vi "MPS_Mag_Core.vi"(0 "EmptyBoreBaseline_Mag_BMon":dbl[](array[numeric])=array[420000 elements], 5 "EmptyBoreBaseline_Mag":dbl[](array[numeric])=array[420000 elements]) -> (1 "Samples Per Acquisition":dbl=21000.0, 3 "Drive IMon":waveform(dbl), 4 "Susceptibility Curves":cluster{"Y":dbl[], "Y":dbl[]}[](graph), 6 "Rx Smooth":dbl[](graph), 10 "BMon_Smooth":dbl[](graph), 12 "Bias Current":waveform(dbl)(graph)={"t0"=timestamp(3727906504.0247726 s since 1904-01-01), "dt"=9.9999999999997e-07, "Y"=array[420000 elements], "attributes"=variant("NI_ChannelName"=variant(string "H1/ai5"), "NI_UnitDescription"=variant(string "Volts"))}, 13 "Rx_Raw":waveform(dbl), 14 "RxBaselineSub":waveform(dbl)(graph), 15 "Bias Smooth":dbl[](graph))   [LabVIEW 2021]
uses:
  <vilib>/Analysis/baseanly.llb/Mean (DBL).vi
  <extravilib>/ChannelInstances/Tag-dbl/Write With Abort.vi
  MPS_global_variables.vi
  <extravilib>/ChannelInstances/Tag-dbl/Instantiate.vi
  <extravilib>/ChannelInstances/Tag-dbl/Endpoint.vi
  <extravilib>/ChannelInstances/Tag-dbl.lvlib
  <vilib>/Analysis/NI_AALBase.lvlib
panel:
  out "Bias Current Amps":waveform(dbl)(graph)={"t0"=timestamp(3727906504.0247726 s since 1904-01-01), "dt"=9.9999999999997e-07, "Y"=array[420000 elements], "attributes"=variant("NI_ChannelName"=variant(string "H1/ai5"), "NI_UnitDescription"=variant(string "Volts"))}
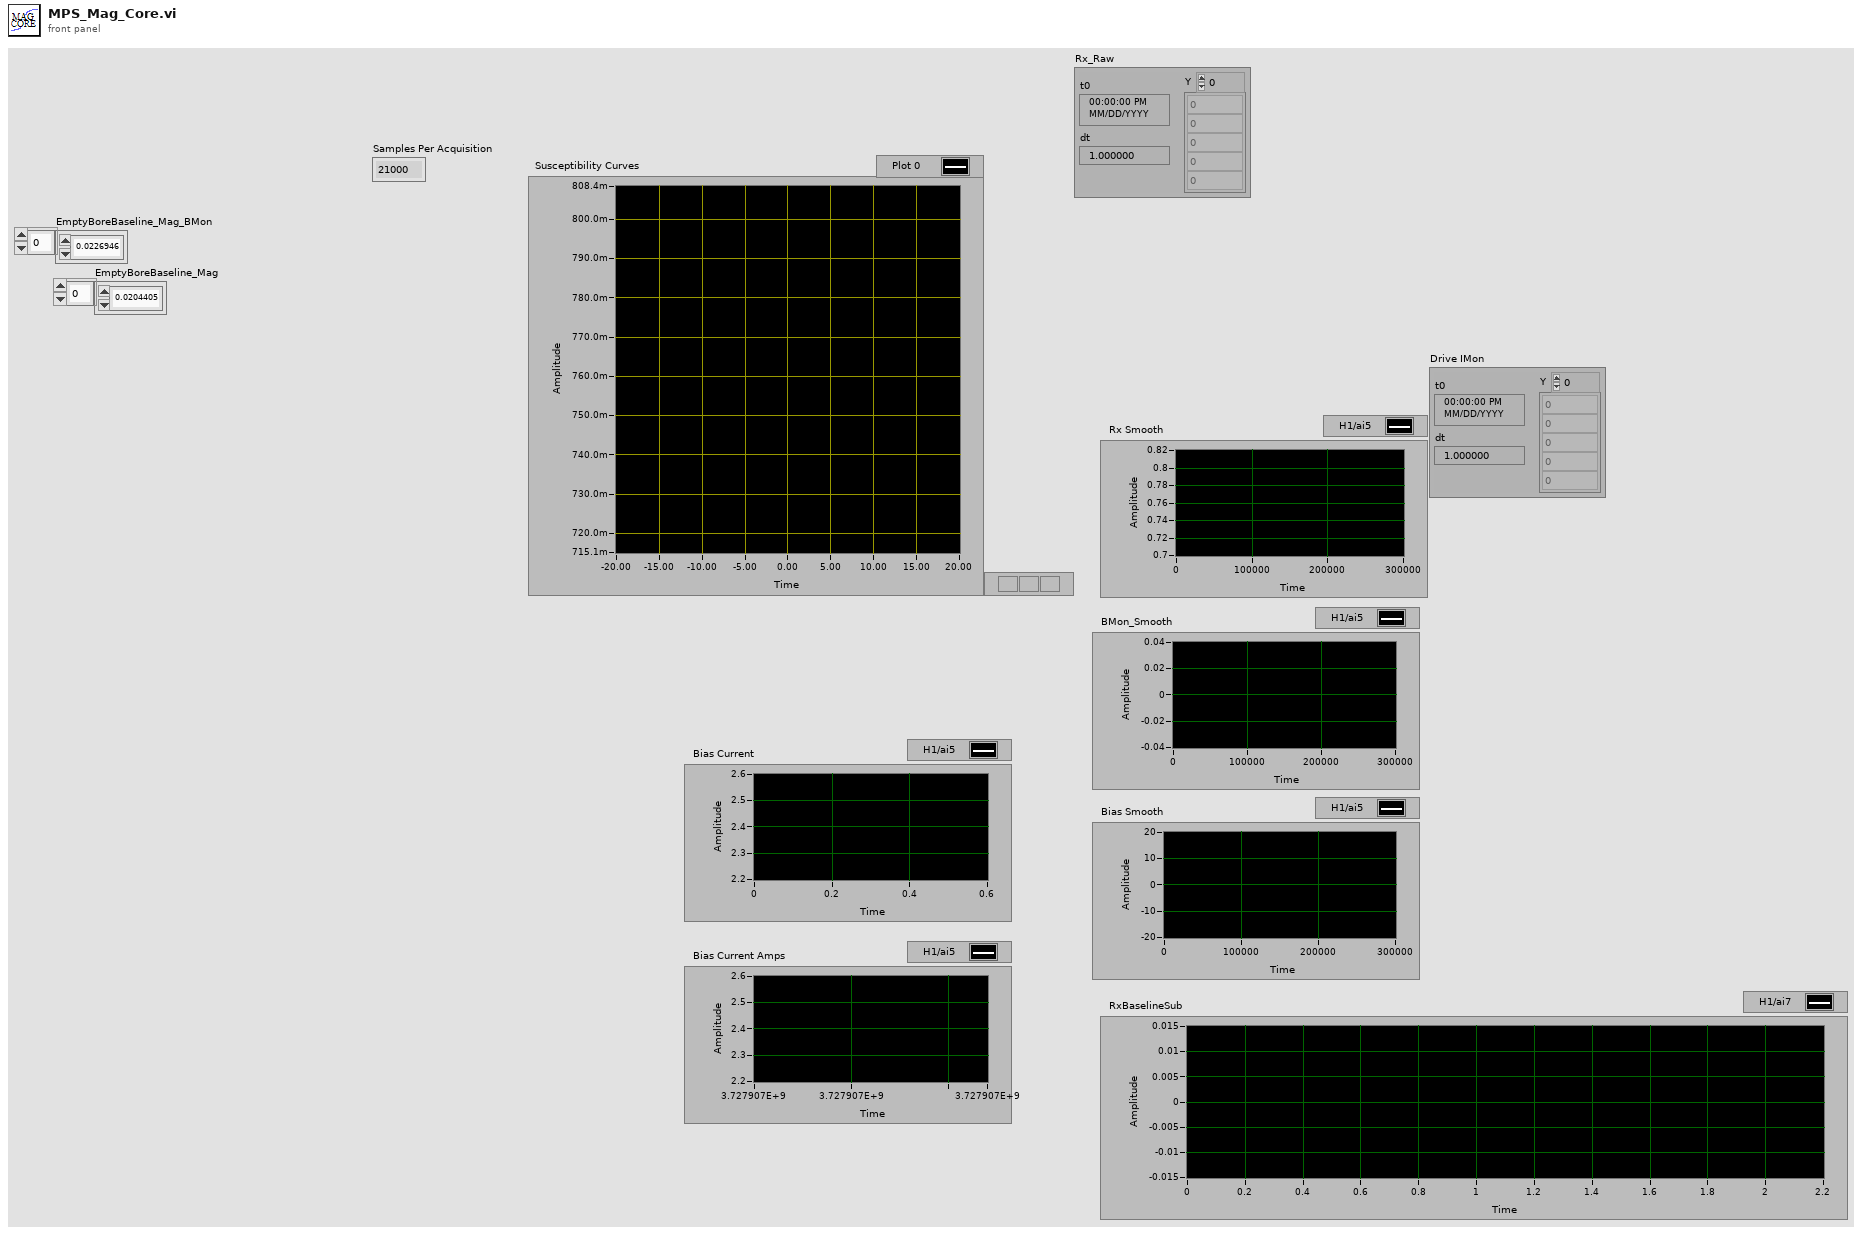
[diagram p1: front panel]
types:
  T1 = typedef "Tag-dbl.lvlib/))Channel.ctl" = refnum<queue>
  T2 = cluster{"sample rate":dbl, "Tx freq":dbl, "Tx amp":dbl, "Tx cycles\nSpectroscopy":dbl, "Bias amp":dbl, "Bias freq":dbl, "Receive range":dbl, "Bias Periods\nMagnetometry":dbl, "Tx Freq Division Factor":dbl, "Drive Periods per Bias":dbl, "TX harmonics":dbl[]}
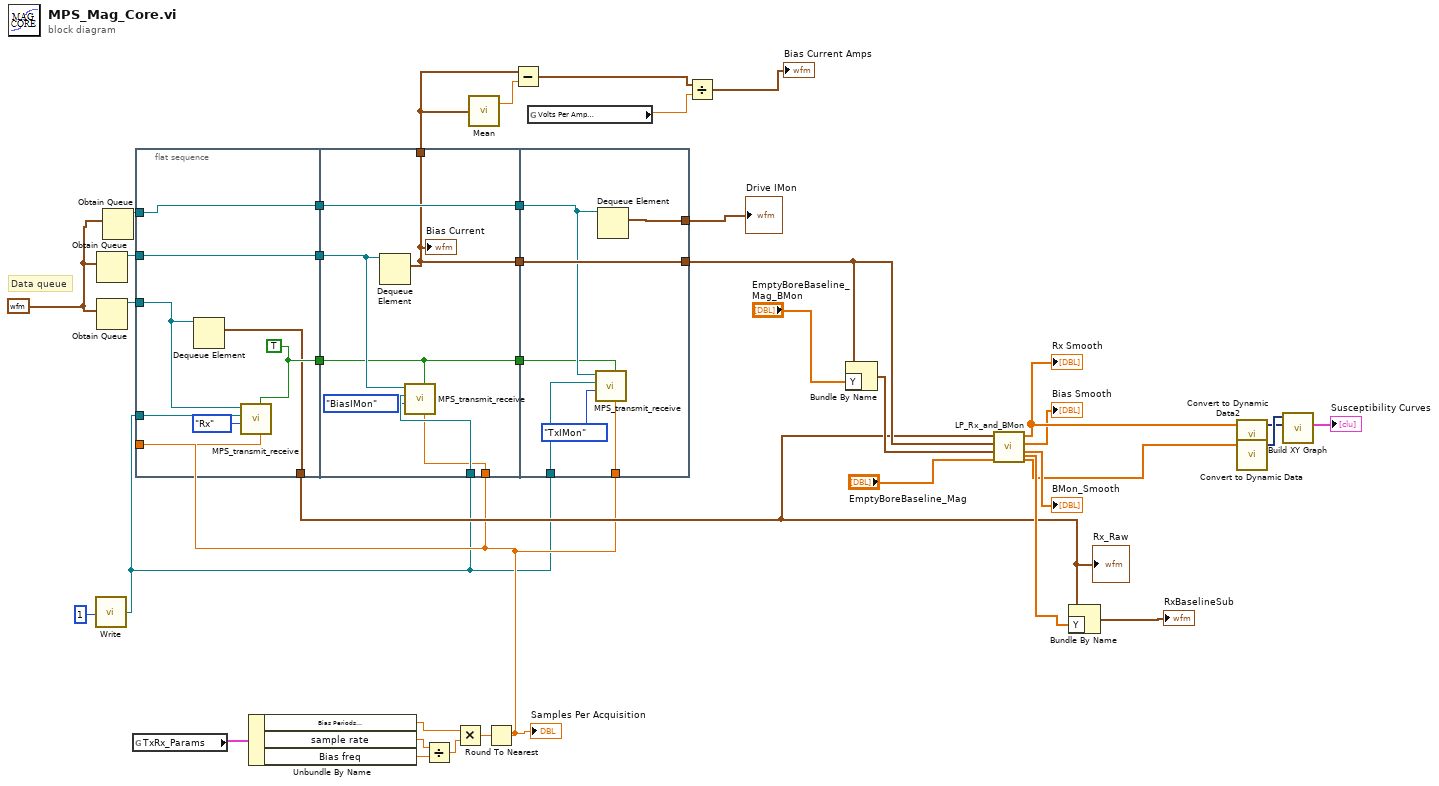
[diagram p0: block diagram]
diagram:
  w14 = waveform(dbl) {"t0"=timestamp(0 s since 1904-01-01), "dt"=1.0, "Y"=[]} ("Waveform")
  # "Data queue"
  n1 = call <extravilib>:"Write.vi"("element"=1 ("number of readouts")) -> ("channel"=w8:T1)  [unwired: 1 out]
  n2 = Obtain Queue(element data type=w14) -> (queue out=w35:refnum<queue>)  [unwired: 4 in, 2 out]
  n3 = Obtain Queue(element data type=w14) -> (queue out=w36:refnum<queue>)  [unwired: 4 in, 2 out]
  n4 = Obtain Queue(element data type=w14) -> (queue out=w11:refnum<queue>)  [unwired: 4 in, 2 out]
  n5 = global read "MPS_global_variables.vi" "TxRx_Params"() -> (w29:T2)
  n6 = flat-sequence {
    tunnel: w36 -> [w46]
    tunnel: [w45] -> w39
    tunnel: w8 -> [w47]
    tunnel: w35 -> [w45]
    tunnel: [w42] -> w16
    tunnel: w9 -> [w44]
    tunnel: [w43] -> w38
    tunnel: [w41] -> w12
    tunnel: w11 -> [w41]
    tunnel: w39 -> [w54]
    tunnel: w8 -> [w53]
    tunnel: w9 -> [w52]
    tunnel: w38 -> [w49]
    tunnel: [w48] -> w15
    tunnel: [w51] -> w13
    tunnel: w12 -> [w51]
    tunnel: [w49] -> w7
    tunnel: [w48] -> w4
    tunnel: [w61] -> w22
    tunnel: w15 -> [w61]
    tunnel: w13 -> [w59]
    tunnel: [w60] -> w10
    tunnel: w9 -> [w57]
    tunnel: w8 -> [w56]
    tunnel: w7 -> [w55]
    frame #0 {
      w43 = TRUE ("Use Bias? 5")
      n7 = Dequeue Element(queue=w46) -> (element=w42:waveform(dbl))  [unwired: 2 in, 3 out]
      n8 = call "MPS_transmit_receive.vi"("samples per readout"=w44, "Use Bias?"=w43, "InputChans"=enum16{"Rx", "BiasIMon", "TxIMon", "BMon"}."Rx", "channel input for max readouts"=w47, "Measurement Queue"=w46) -> ()  [unwired: 7 in]
    }
    frame #1 {
      n9 = Dequeue Element(queue=w54) -> (element=w48:waveform(dbl))  [unwired: 2 in, 3 out]
      "Bias Current" <- w48
      n10 = call "MPS_transmit_receive.vi"("samples per readout"=w52, "Use Bias?"=w49, "InputChans"=enum16{"Rx", "BiasIMon", "TxIMon", "BMon"}."BiasIMon", "channel input for max readouts"=w53, "Measurement Queue"=w54) -> ()  [unwired: 7 in]
    }
    frame #2 {
      n11 = call "MPS_transmit_receive.vi"("samples per readout"=w57, "Use Bias?"=w55, "InputChans"=enum16{"Rx", "BiasIMon", "TxIMon", "BMon"}."TxIMon", "channel input for max readouts"=w56, "Measurement Queue"=w59) -> ()  [unwired: 7 in]
      n12 = Dequeue Element(queue=w59) -> (element=w60:waveform(dbl))  [unwired: 2 in, 3 out]
    }
  }
  n13 = Unbundle By Name(w29) -> ("Bias Periods\nMagnetometry"=w25:dbl, "sample rate"=w28:dbl, "Bias freq"=w27:dbl)
  n14 = Divide(x=w28, y=w27) -> (x/y=w26:dbl)
  n15 = Multiply(x=w25, y=w26) -> (x*y=w24:dbl)
  n16 = call-poly <vilib>:"Mean.vi"("X"=w4) -> ("mean"=w5:dbl)  [unwired: 1 out]
  n17 = Round To Nearest(number=w24) -> (nearest integer value=w9:dbl)
  "Samples Per Acquisition" <- w9
  n18 = Subtract(x=w4, y=w5) -> (x-y=w2:waveform(dbl))
  n19 = global read "MPS_global_variables.vi" "Volts Per Amp\nBias"() -> (w3:dbl)
  n20 = Divide(x=w2, y=w3) -> (x/y=→"Bias Current Amps":waveform(dbl))
  n21 = Bundle By Name(cluster=w22, "Y"="EmptyBoreBaseline_Mag_BMon") -> (w21:waveform(dbl))
  n22 = call "LP_Rx_and_BMon.vi"("Rx"=w16, "Bias"=w22, "BMon"=w21, "BaselineSig"="EmptyBoreBaseline_Mag") -> ("RxBaselineSub"=w18:dbl[], "RX_Smooth"=w31:dbl[], "BiasSmooth"=→"Bias Smooth":dbl[], "BMon Smooth"=→"BMon_Smooth":dbl[], "Bias Reconstructed"=w6:dbl[])  [unwired: 1 in]
  "Rx Smooth" <- w31
  n23 = Bundle By Name(cluster=w16, "Y"=w18) -> (→"RxBaselineSub":waveform(dbl))
  n24 = call "Convert to Dynamic Data2"("Array"=w31) -> ("Dynamic Data Type"=w32:dynamicdata)  [unwired: 3 in]
  n25 = call "Convert to Dynamic Data"("Array"=w6) -> ("Dynamic Data Type"=w33:dynamicdata)  [unwired: 3 in]
  n26 = call "Build XY Graph"("Y Input"=w32, "X Input"=w33) -> ("XY Graph"=→"Susceptibility Curves":cluster{"X":dbl[], "Y":dbl[]}[])  [unwired: 8 in, 1 out]
  "Drive IMon" <- w10
  "Rx_Raw" <- w16
